vi "cropAndSave.vi"(0 "Particle Measurements (Pixels)":dbl[][](array[numeric]) format="%.2f", 1 "Number of Particles":i32, 3 "cropped Image":T1, 4 "std threshold":sgl, 5 "raw image":T1=refnum, 9 "processed image":T1=refnum, 10 "downsampling":i32, 11 "Standard Variation":sgl, 12 "buffer number":u32, 14 "error in":errorcluster) -> (6 "error out":errorcluster, 8 "raw image out":T1, 15 "cropped image out":T1)   [LabVIEW 2012]
uses:
  <vilib>/vision/Image Controls.llb/IMAQ Image.ctl
  GlobalBaslerCamera.vi
  <vilib>/imath/engines/lvmath2/RunTimeEngine/ErrorHandling/NIMS_Finalize Error.vi
  <vilib>/imath/engines/lvmath2/RunTimeEngine/NodeEndStatement/NIMS_NodeEndStatement_Output.vi
  <instcachedir>/0/NIMS_NodeEndStatement_Output_53EC0D466D134D7ABD903AC30B43404B.lvgen/NIMS_NodeEndStatement_Output_53EC0D466D134D7ABD903AC30B43404B_004.vi
  <vilib>/imath/engines/lvmath2/RunTimeEngine/RangeToken/NIMS_Range_R2.vi
  <vilib>/imath/engines/lvmath2/RunTimeEngine/VariableToken/Read/NIMS_Get Elements - SorM(_) - Check.vi
  <instcachedir>/0/NIMS_Get Elements - SorM(_) - Check_8FDA2664A675493882C25203DD903B51.lvgen/NIMS_Get Elements - SorM(_) - Check_8FDA2664A675493882C25203DD903B51_001.vi
  <vilib>/imath/engines/lvmath2/RunTimeEngine/BuiltInFunctions/round/NIMS_round(DBL-M).vi
  <vilib>/imathl/engines/lvmath/Functions/Error Handling/Create Error.vi
  <instcachedir>/0/NIMS_Get Elements - SorM(_) - Check_8FDA2664A675493882C25203DD903B51.lvgen/NIMS_Get Elements - SorM(_) - Check_8FDA2664A675493882C25203DD903B51_000.vi
  <vilib>/imath/engines/lvmath2/RunTimeEngine/ReplaceToken/NIMS_Replace - Check Linear.vi
  <instcachedir>/0/NIMS_Replace - Check Linear_44ABB4D6A819426DBDF25CCE6827BF1D.lvgen/NIMS_Replace - Check Linear_44ABB4D6A819426DBDF25CCE6827BF1D_001.vi
  <vilib>/imath/engines/lvmath2/RunTimeEngine/ReplaceToken/NIMS_Replace - Size Check _(_)=S.vi
  <instcachedir>/0/NIMS_Replace - Size Check _(_)=S_5AC8AA27B9694BB9828B57BCF666F597.lvgen/NIMS_Replace - Size Check _(_)=S_5AC8AA27B9694BB9828B57BCF666F597_000.vi
  <vilib>/imath/engines/lvmath2/RunTimeEngine/ReplaceToken/NIMS_Replace - V(S)=S.vi
  <instcachedir>/0/NIMS_Replace - V(S)=S_927EF1B21AA84780A9A306EC96B904EC.lvgen/NIMS_Replace - V(S)=S_927EF1B21AA84780A9A306EC96B904EC_000.vi
  <vilib>/imath/engines/lvmath2/RunTimeEngine/ErrorHandling/NIMS_Create Error From Enums.vi
  <instcachedir>/0/NIMS_Replace - Check Linear_44ABB4D6A819426DBDF25CCE6827BF1D.lvgen/NIMS_Replace - Check Linear_44ABB4D6A819426DBDF25CCE6827BF1D_008.vi
  <instcachedir>/0/NIMS_Replace - Size Check _(_)=S_5AC8AA27B9694BB9828B57BCF666F597.lvgen/NIMS_Replace - Size Check _(_)=S_5AC8AA27B9694BB9828B57BCF666F597_007.vi
  <instcachedir>/0/NIMS_Replace - V(S)=S_927EF1B21AA84780A9A306EC96B904EC.lvgen/NIMS_Replace - V(S)=S_927EF1B21AA84780A9A306EC96B904EC_003.vi
  <vilib>/Utility/file.llb/Write To Spreadsheet File (I64).vi
  daq test/GlobalStatus.vi
  <vilib>/vision/NI_Vision_Development_Module.lvlib
  <resource>/objmgr/IMAQImage.rc
panel:
  out "Image Size":cluster{"x":i32, "y":i32}
  out "out of focus":bool
  out "saving to disk":bool
  out "touching borders":bool
  in  "cropHeight":i32=600
  in  "cropWidth":i32=1200
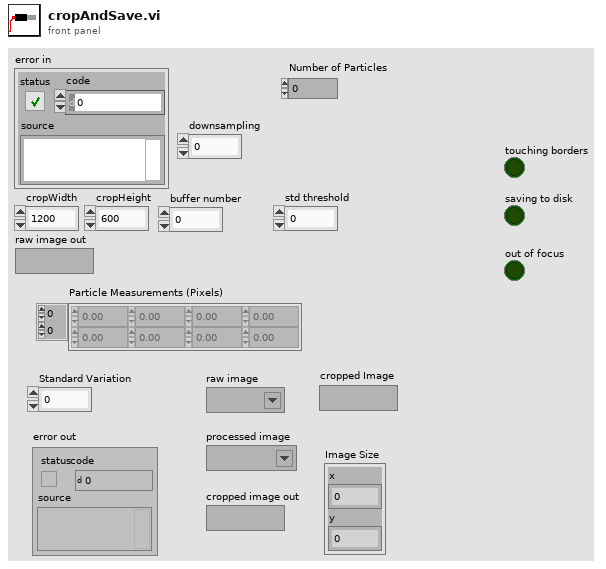
[diagram p1: front panel]
types:
  T1 = typedef "IMAQ Image.ctl" = refnum<image>
  T2 = cluster{"rectangle[0]":i32, "rectangle[1]":i32, "rectangle[2]":i32, "rectangle[3]":i32}
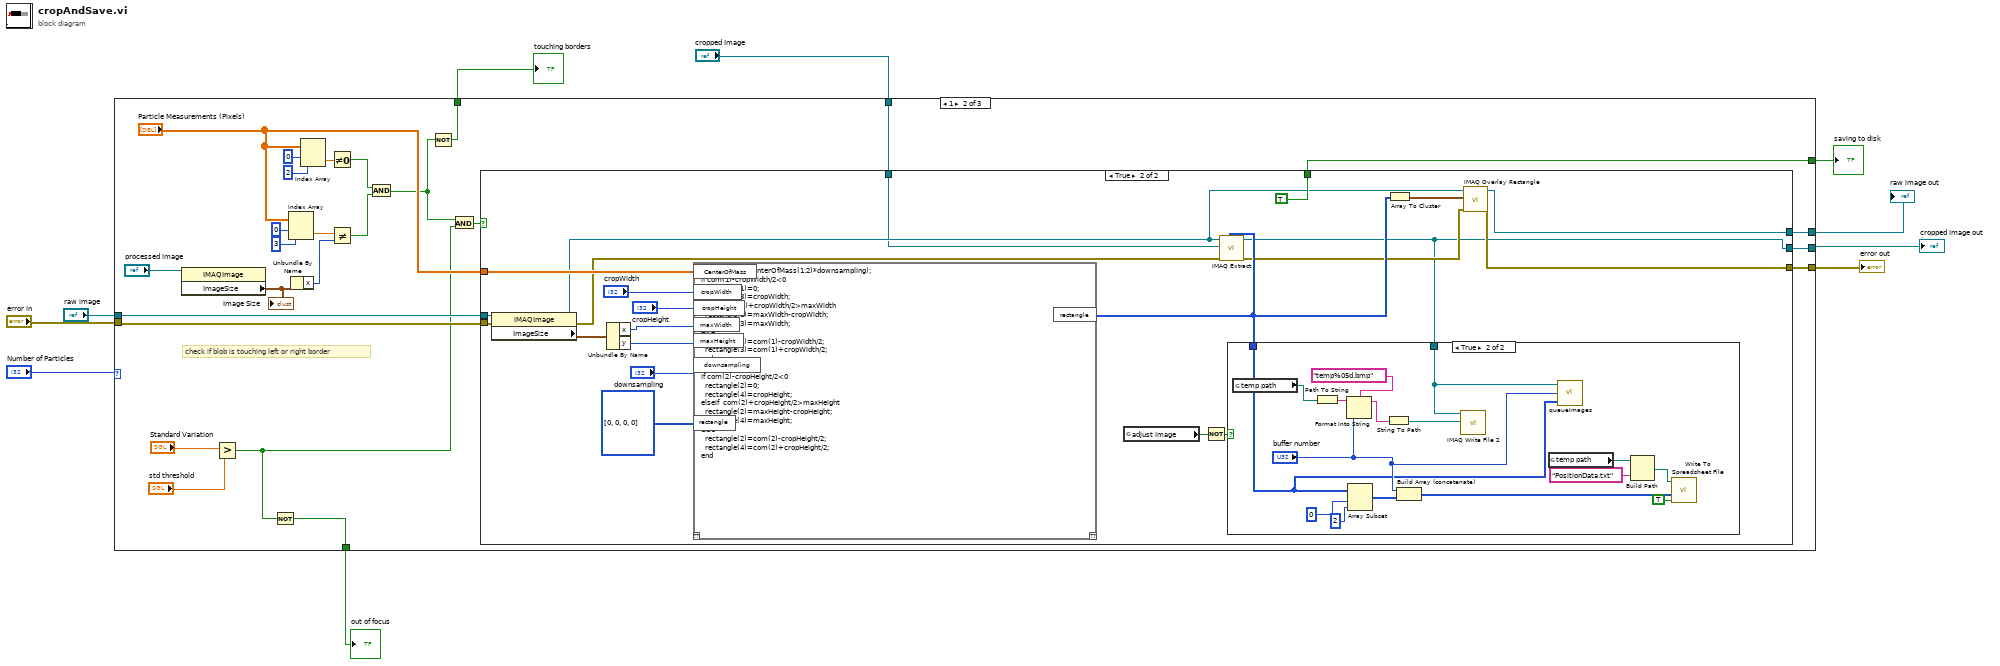
[diagram p0: block diagram]
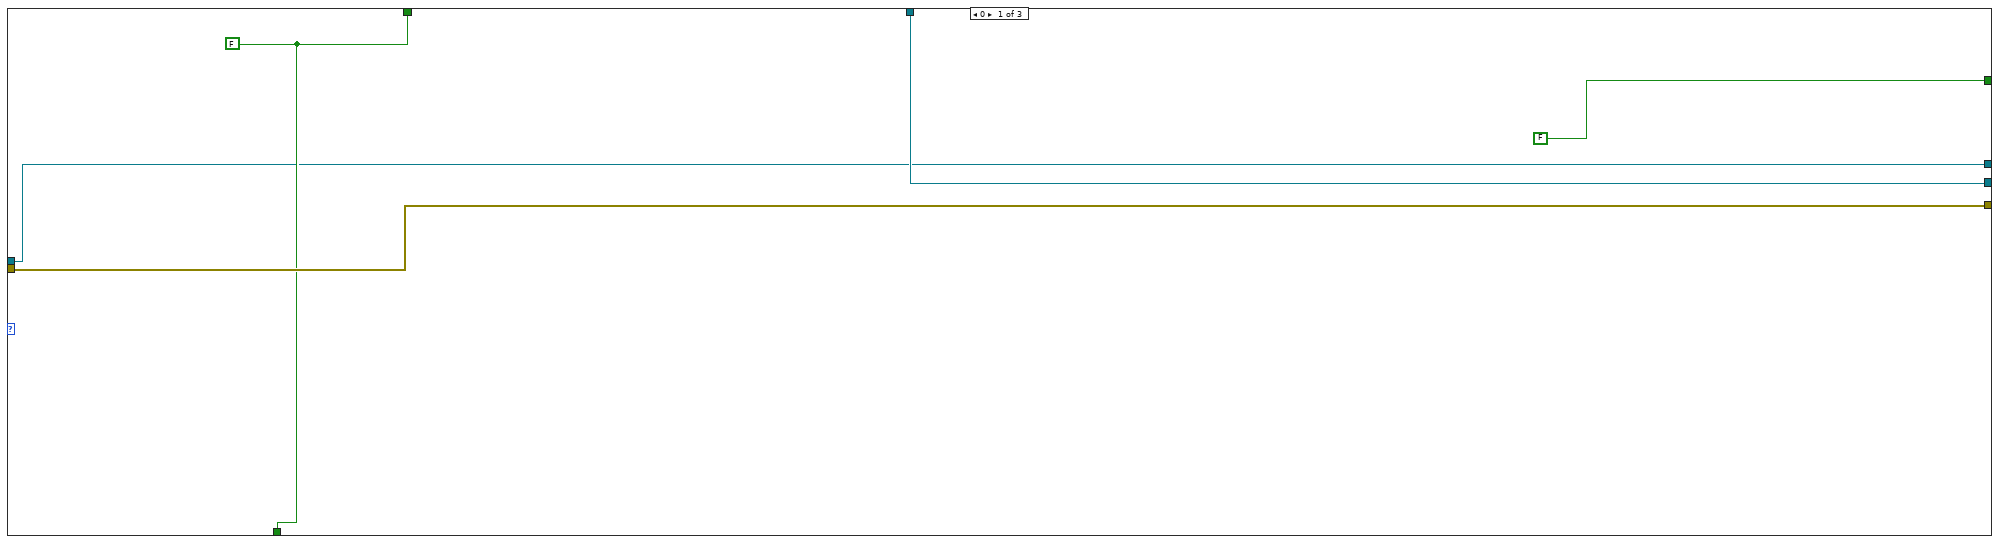
[diagram p2: hidden frame]
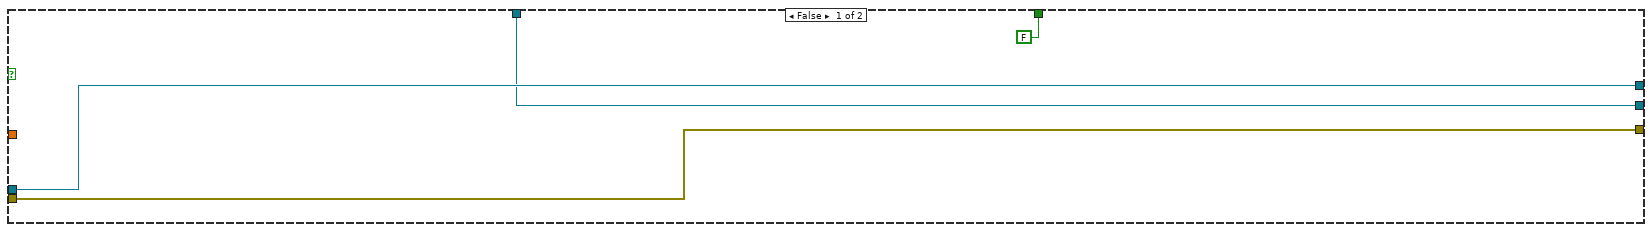
[diagram p3: hidden frame]
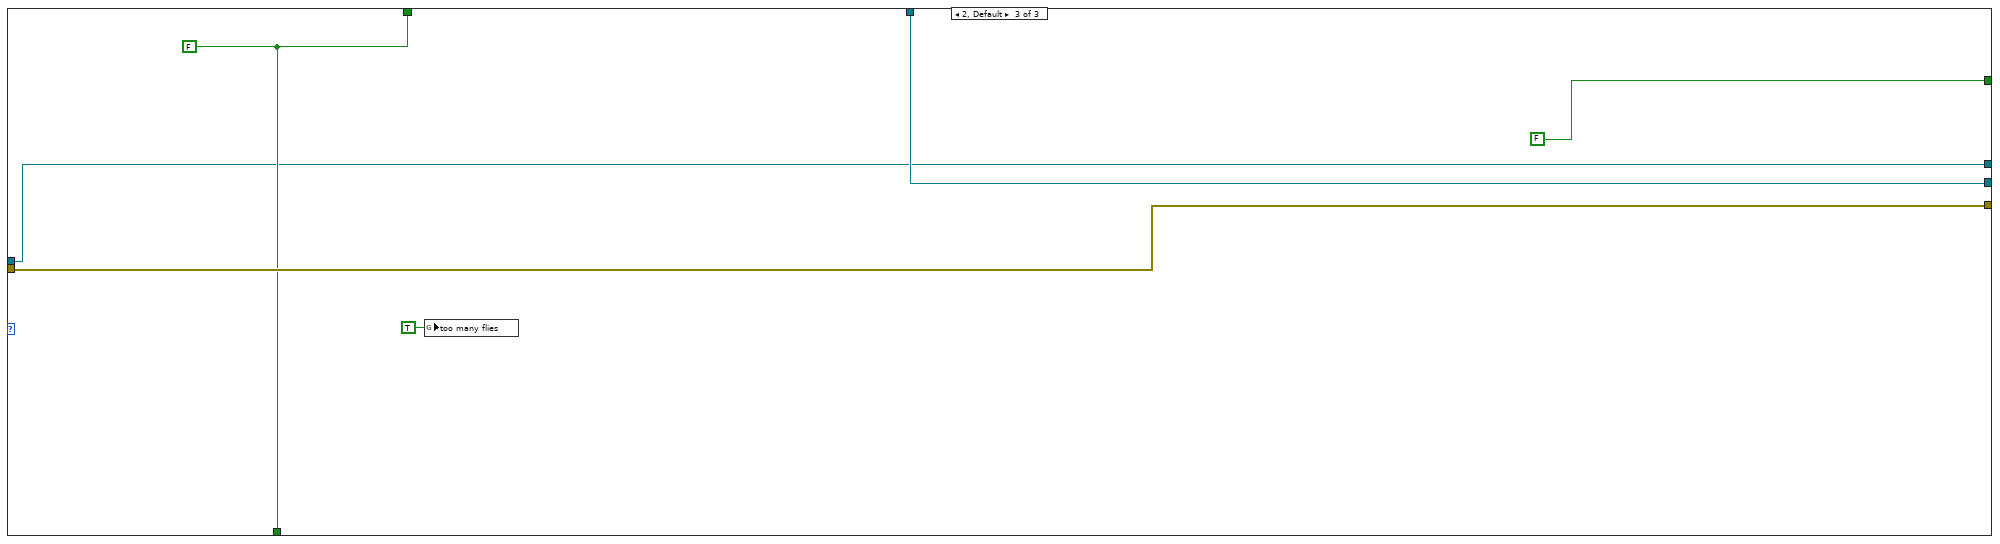
[diagram p5: hidden frame]
diagram:
  n1 = case shown="1" "Number of Particles" {
    tunnel: "error in" -> [w15 w31 w495]
    tunnel: "raw image" -> [w11 w32 w490]
    tunnel: [w15 w41 w495] -> w8
    tunnel: [FALSE w30 FALSE] -> w6
    tunnel: [w13 w27 w492] -> w5
    tunnel: [w13 w25 w492] -> w4
    tunnel: [w12 w16 w491] -> w1
    tunnel: "cropped Image" -> [w12 w18 w491]
    tunnel: [w11 w17 w490] -> w2
    frame 0 {
      w13 = FALSE
    }
    frame 1 {
      # "check if blob is touching left or right border"
      n2 = property class="IMAQImage"(reference="processed image") -> ("ImageSize"=w33:cluster{"x":i32, "y":i32})  [unwired: 1 in, 2 out]
      "Image Size" <- w33
      n3 = Greater?(x="Standard Variation", y="std threshold") -> (0:w24:bool)
      n4 = Not(x=w24) -> (.not. x?=w25:bool)
      n5 = Index Array(array="Particle Measurements (Pixels)", index (row)=0, index (col)=3 ("disabled index (col)")) -> (element=w23:dbl)
      n6 = Unbundle By Name(w33) -> ("x"=w22:i32)
      n7 = Index Array(array="Particle Measurements (Pixels)", index (row)=0, index (col)=2 ("disabled index (col)")) -> (element=w39:dbl)
      n8 = Not Equal To 0?(x=w39) -> (x != 0?=w21:bool)
      n9 = Not Equal?(x=w23, y=w22) -> (x != y?=w20:bool)
      n10 = And(x=w21, y=w20) -> (x .and. y?=w19:bool)
      n11 = Not(x=w19) -> (.not. x?=w27:bool)
      n12 = And(x=w19, y=w24) -> (x .and. y?=w26:bool)
      n13 = case shown="True" w26 {
        tunnel: w32 -> [w43 w59]
        tunnel: [w45 w49] -> w41
        tunnel: "Particle Measurements (Pixels)" -> [_ w64]
        tunnel: w31 -> [w45 w58]
        tunnel: [FALSE TRUE] -> w30
        tunnel: w18 -> [w42 w52]
        tunnel: [w43 w51] -> w17
        tunnel: [w42 w48] -> w16
        frame False {
        }
        frame True {
          n14 = property class="IMAQImage"(reference=w59, error in=w58) -> (reference out=w53:T1, error out=w60:errorcluster, "ImageSize"=w62:cluster{"x":i32, "y":i32})
          n15 = Unbundle By Name(w62) -> ("x"=w63:i32, "y"=w61:i32)
          n16 = mathscript code="com = round(CenterOfMass(1:2)*downsampling);\nif com(1)-cropWidth/2<0\n  rectangle(1)=0;\n  rectangle(3)=cropWidth;\nelseif  com(1)+cropWidth/2>maxWidth\n  rectangle(1)=maxWidth-cropWidth;\n  rectangle(3)=maxWidth;\nelse\n  rectangle(1)=com(1)-cropWidth/2;\n  rectangle(3)=com(1)+cropWidth/2;\nend\n\nif com(2)-cropHeight/2<0\n  rectangle(2)=0;\n  rectangle(4)=cropHeight;\nelseif  com(2)+cropHeight/2>maxHeight\n  rectangle(2)=maxHeight-cropHeight;\n  rectangle(4)=maxHeight;\nelse\n  rectangle(2)=com(2)-cropHeight/2;\n  rectangle(4)=com(2)+cropHeight/2;\nend"("CenterOfMass"=w64, "cropWidth"="cropWidth", "maxWidth"=w63, "maxHeight"=w61, "cropHeight"="cropHeight", "downsampling"="downsampling", "rectangle"=i32[] [0, 0, 0, 0]) -> ("rectangle"=w54:i32[])  [unwired: 1 in, 1 out]
          n17 = global read "GlobalBaslerCamera.vi" "adjust image"() -> (w47:bool)
          n18 = Not(x=w47) -> (.not. x?=w46:bool)
          n19 = call "IMAQ Extract"("Optional Rectangle"=w54, "error in (no error)"=w60, "Image Dst"=w52, "Image Src"=w53) -> ("error out"=w50:errorcluster, "Image Dst Out"=w48:T1)  [unwired: 6 in]
          n20 = case shown="True" w46 {
            tunnel: w54 -> [_ w68]
            tunnel: w48 -> [_ w70]
            frame False {
            }
            frame True {
              n21 = global read "GlobalBaslerCamera.vi" "temp path"() -> (w71:path)
              n22 = Path To String(path=w71) -> (string=w72:string)
              n23 = Format Into String(format string="temp%05d.bmp", initial string=w72, "buffer number") -> (resulting string=w83:string)  [unwired: 1 in, 1 out]
              n24 = Array Subset(array=w68, index=0, length=2) -> (w79:i32[])
              n25 = String To Path(string=w83) -> (path=w82:path)
              n26 = Build Array (concatenate)("buffer number", w79) -> (w77:u32[])
              n27 = call-poly "IMAQ Write File 2"("File Path"=w82, "Image"=w70) -> ()  [unwired: 8 in, 2 out]
              n28 = global read "GlobalBaslerCamera.vi" "temp path"() -> (w75:path)
              n29 = call "queueImages.vi"("rectangle"=w68, "buffer number"="buffer number", "Image Src"=w70) -> ()
              n30 = Build Path(base path=w75, name or relative path="PositionData.txt") -> (appended path=w73:path)
              n31 = call-poly <vilib>:"Write To Spreadsheet File.vi"("append to file? (new file:F)"=TRUE, "1D data"=w77, "file path (dialog if empty)"=w73) -> ()  [unwired: 5 in, 1 out]
            }
          }
          n32 = Array To Cluster(array=w54) -> (cluster=w55:T2)
          n33 = call "IMAQ Overlay Rectangle"("error in (no error)"=w50, "Rectangle"=w55, "Image"=w53) -> ("error out"=w49:errorcluster, "Image Out"=w51:T1)  [unwired: 7 in]
        }
      }
    }
    frame 2, Default {
      w492 = FALSE
      n34 = global write "GlobalStatus.vi" "too many flies"(TRUE ("too many flies")) -> ()
    }
  }
  "error out" <- w8
  "touching borders" <- w5
  "saving to disk" <- w6
  "out of focus" <- w4
  "cropped image out" <- w1
  "raw image out" <- w2
